vi "TLB Native Dynamic Events ver 0.25.vi"() -> ()   [LabVIEW 2018] (continued)
              tunnel: [w613 State_Type_Definitions."True Stop" ("Enum")] -> w597
              tunnel: [w611 w628] -> w590
              tunnel: w599 -> [w610 _]
              tunnel: w598 -> [w604 _]
              tunnel: [State_Type_Definitions."Idle" ("Enum") State_Type_Definitions."Shutdown" ("Enum")] -> w596
              tunnel: w600 -> [w603 _]
              frame "Start Task 1", Default {
                # ">> WIill proceed to part ii if not manual override >>"
                # ">>If ENABLE or Trigger is set to true>>"
                n263 = Or(x=w603, y=w604) -> (x .or. y?=w605:bool)
                n264 = case shown="True" w603 {
                  tunnel: [w616 w622] -> w611
                  tunnel: w610 -> [w615 w621]
                  frame False {
                    n265 = for {
                      shift-right: [w618] -> w616
                      shift-left: w615 -> [w619]
                      tunnel: string[] ["Z STEPPER CAM HEIGHT", "READ STEPPER VALUES"] ("element") -> [w617] mode=indexing
                      n266 = Enqueue Element(queue=w619, element=w617) -> (queue out=w618:refnum<queue>)  [unwired: 2 in, 2 out]
                    }
                  }
                  frame True {
                    n267 = for {
                      shift-right: [w624] -> w622
                      shift-left: w621 -> [w625]
                      tunnel: string[] ["ARDUINO - ULTRASONIC", "READ ULTRASONIC", "", "", "", ""] -> [w623] mode=indexing
                      n268 = Enqueue Element(queue=w625, element=w623) -> (queue out=w624:refnum<queue>)  [unwired: 2 in, 2 out]
                    }
                  }
                }
                n269 = Select(t=State_Type_Definitions."True Stop" ("Enum"), s=w604, f=State_Type_Definitions."Task 2:Sensor Mode" ("Enum")) -> (s? t:f=w607:T16)
                n270 = Select(t=w607, s=w605, f=State_Type_Definitions."Task 2:Raise Arm" ("Enum")) -> (s? t:f=w613:T16)
              }
              frame "Exit" {
                n271 = for {
                  shift-right: [w631] -> w628
                  shift-left: _ -> [w632]
                  tunnel: string[] ["STOP", "RESET ENCODERS", "RESET YAW", ""] -> [w630] mode=indexing
                  n272 = Enqueue Element(queue=w632, element=w630) -> (queue out=w631:refnum<queue>)  [unwired: 2 in, 2 out]
                }
              }
            }
          }
          frame "Task 2:Sensor Mode" {
            w649 = u8 20 ("y")
            # ">>> yStepper command>>>"
            # ">>Object detected>>"
            n273 = Dequeue Element(queue=w642, timeout in ms (-1)=w641, error in (no error)=w640) -> (element=w650:T8)  [unwired: 3 out]
            n274 = Less?(x=w638, y=w649) -> (x < y?=w648:bool)
            n275 = Less?(x=w637, y=w649) -> (x < y?=w647:bool)
            n276 = Or(x=w648, y=w647) -> (x .or. y?=w633:bool)
            n277 = case shown="\"Start Task 1\", Default" w650 {
              tunnel: w633 -> [w653 _]
              tunnel: [w660 State_Type_Definitions."True Stop" ("Enum")] -> w646
              tunnel: w639 -> [w652 _]
              tunnel: w643 -> [w659 w676]
              tunnel: [w658 w677] -> w645
              tunnel: [State_Type_Definitions."Idle" ("Enum") State_Type_Definitions."Shutdown" ("Enum")] -> w644
              frame "Start Task 1", Default {
                n278 = case shown="False" w653 {
                  tunnel: w659 -> [w663 w670]
                  tunnel: [w664 w669] -> w658
                  frame False {
                    n279 = for {
                      tunnel: string[] ["READ ULTRASONIC", "STOP"] ("element") -> [w665] mode=indexing
                      shift-right: [w667] -> w664
                      shift-left: w663 -> [w666]
                      n280 = Enqueue Element(queue=w666, element=w665) -> (queue out=w667:refnum<queue>)  [unwired: 2 in, 2 out]
                    }
                  }
                  frame True {
                    n281 = for {
                      shift-right: [w672] -> w669
                      shift-left: w670 -> [w673]
                      tunnel: string[] ["RESET ENCODERS", "READ NAVX", "READ ENCODERS"] -> [w671] mode=indexing
                      n282 = Enqueue Element(queue=w673, element=w671) -> (queue out=w672:refnum<queue>)  [unwired: 2 in, 2 out]
                    }
                  }
                }
                n283 = Or(x=w653, y=w652) -> (x .or. y?=w651:bool)
                n284 = Select(t=State_Type_Definitions."True Stop" ("Enum"), s=w652, f=State_Type_Definitions."Task 2:Reverse Mode" ("Enum")) -> (s? t:f=w654:T16)
                n285 = Select(t=w654, s=w651, f=State_Type_Definitions."Task 2:Sensor Mode" ("Enum")) -> (s? t:f=w660:T16)
              }
              frame "Exit" {
                n286 = for {
                  shift-right: [w680] -> w677
                  shift-left: w676 -> [w681]
                  tunnel: string[] ["STOP", "RESET ENCODERS", "RESET YAW", "ARDUINO MODE 0"] -> [w679] mode=indexing
                  n287 = Enqueue Element(queue=w681, element=w679) -> (queue out=w680:refnum<queue>)  [unwired: 2 in, 2 out]
                }
              }
            }
          }
          frame "Task 2:Reverse Mode" {
            # ">>> yStepper command>>>"
            n288 = Dequeue Element(queue=w692, timeout in ms (-1)=w693, error in (no error)=w694) -> (element=w696:T8)  [unwired: 3 out]
            n289 = Less?(x=w686, y=-50.0) -> (x < y?=w684:bool)
            n290 = case shown="\"Start Task 1\", Default" w696 {
              tunnel: [w706 State_Type_Definitions."True Stop" ("Enum")] -> w688
              tunnel: w695 -> [w699 _]
              tunnel: w691 -> [w705 w722]
              tunnel: [w704 w723] -> w687
              tunnel: [State_Type_Definitions."Idle" ("Enum") State_Type_Definitions."Shutdown" ("Enum")] -> w689
              tunnel: w684 -> [w697 _]
              frame "Start Task 1", Default {
                n291 = case shown="True" w697 {
                  tunnel: w705 -> [w709 w716]
                  tunnel: [w710 w715] -> w704
                  frame False {
                    n292 = for {
                      tunnel: string[] ["READ ENCODERS", "REVERSE", "READ NAVX"] ("element") -> [w711] mode=indexing
                      shift-right: [w713] -> w710
                      shift-left: w709 -> [w712]
                      n293 = Enqueue Element(queue=w712, element=w711) -> (queue out=w713:refnum<queue>)  [unwired: 2 in, 2 out]
                    }
                  }
                  frame True {
                    n294 = for {
                      shift-right: [w718] -> w715
                      shift-left: w716 -> [w719]
                      tunnel: string[] ["STOP", "ARDUINO - ULTRASONIC", "READ ULTRASONIC", "RESET ENCODERS"] -> [w717] mode=indexing
                      n295 = Enqueue Element(queue=w719, element=w717) -> (queue out=w718:refnum<queue>)  [unwired: 2 in, 2 out]
                    }
                  }
                }
                n296 = Or(x=w697, y=w699) -> (x .or. y?=w698:bool)
                n297 = Select(t=State_Type_Definitions."True Stop" ("Enum"), s=w699, f=State_Type_Definitions."Task 2:Sensor Mode" ("Enum")) -> (s? t:f=w700:T16)
                n298 = Select(t=w700, s=w698, f=State_Type_Definitions."Task 2:Reverse Mode" ("Enum")) -> (s? t:f=w706:T16)
              }
              frame "Exit" {
                n299 = for {
                  shift-right: [w726] -> w723
                  shift-left: w722 -> [w727]
                  tunnel: string[] ["STOP", "RESET ENCODERS", "RESET YAW", "ARDUINO MODE 0"] -> [w725] mode=indexing
                  n300 = Enqueue Element(queue=w727, element=w725) -> (queue out=w726:refnum<queue>)  [unwired: 2 in, 2 out]
                }
              }
            }
          }
          frame "Task 3" {
            # ">>> Motor control cluster >>>"
            # ">>> yStepper command>>>"
            n301 = Dequeue Element(queue=w743, timeout in ms (-1)=w742, error in (no error)=w741) -> (element=w732:T8)  [unwired: 3 out]
            n302 = Less?(x=w740, y=-160.0) -> (x < y?=w737:bool)
            n303 = Or(x=w737, y=w738) -> (x .or. y?=w733:bool)
            n304 = case shown="\"Start Task 1\", Default" w732 {
              tunnel: w733 -> [w746 _]
              tunnel: [w750 State_Type_Definitions."True Stop" ("Enum")] -> w734
              tunnel: w736 -> [w747 w766]
              tunnel: [w745 w765] -> w735
              tunnel: [State_Type_Definitions."Idle" ("Enum") State_Type_Definitions."Shutdown" ("Enum")] -> w731
              frame "Start Task 1", Default {
                n305 = case shown="False" w746 {
                  tunnel: w747 -> [w753 w759]
                  tunnel: [w752 w757] -> w745
                  frame False {
                    n306 = for {
                      shift-right: [w755] -> w752
                      shift-left: w753 -> [w756]
                      tunnel: string[] ["READ ENCODERS", "R-CW"] ("element") -> [w754] mode=indexing
                      n307 = Enqueue Element(queue=w756, element=w754) -> (queue out=w755:refnum<queue>)  [unwired: 2 in, 2 out]
                    }
                  }
                  frame True {
                    n308 = for {
                      shift-right: [w761] -> w757
                      shift-left: w759 -> [w762]
                      tunnel: string[] ["RESET YAW", "RESET ENCODERS", "STOP", "ARDUINO MODE 0"] -> [w760] mode=indexing
                      n309 = Enqueue Element(queue=w762, element=w760) -> (queue out=w761:refnum<queue>)  [unwired: 2 in, 2 out]
                    }
                  }
                }
                n310 = Select(t=State_Type_Definitions."True Stop" ("Enum"), s=w746, f=State_Type_Definitions."Task 3" ("Enum")) -> (s? t:f=w750:T16)
              }
              frame "Exit" {
                n311 = for {
                  shift-right: [w769] -> w765
                  shift-left: w766 -> [w770]
                  tunnel: string[] ["STOP", "RESET ENCODERS", "RESET YAW", ""] -> [w768] mode=indexing
                  n312 = Enqueue Element(queue=w770, element=w768) -> (queue out=w769:refnum<queue>)  [unwired: 2 in, 2 out]
                }
              }
            }
          }
          frame "Task 4_A" {
            # ">> Stepper height reeached >>"
            # ">>> yStepper command>>>"
            # ">> Manual override >>"
            n313 = Dequeue Element(queue=w784, timeout in ms (-1)=w783, error in (no error)=w782) -> (element=w781:T8)  [unwired: 3 out]
            n314 = Equal?(x=w775, y=u8 60) -> (x = y?=w773:bool)
            n315 = case shown="\"Start Task 1\", Default" w781 {
              tunnel: [w796 State_Type_Definitions."True Stop" ("Enum")] -> w780
              tunnel: [w794 w812] -> w779
              tunnel: w785 -> [w793 w809]
              tunnel: w778 -> [w787 _]
              tunnel: [State_Type_Definitions."Idle" ("Enum") State_Type_Definitions."Shutdown" ("Enum")] -> w777
              tunnel: w773 -> [w786 _]
              frame "Start Task 1", Default {
                # ">> WIill proceed to part ii if not manual override >>"
                # ">>If ENABLE or Trigger is set to true>>"
                n316 = Or(x=w786, y=w787) -> (x .or. y?=w788:bool)
                n317 = case shown="False" w786 {
                  tunnel: [w799 w805] -> w794
                  tunnel: w793 -> [w798 w804]
                  frame False {
                    n318 = for {
                      shift-right: [w801] -> w799
                      shift-left: w798 -> [w802]
                      tunnel: string[] ["Z STEPPER CAM HEIGHT", "READ STEPPER VALUES"] ("element") -> [w800] mode=indexing
                      n319 = Enqueue Element(queue=w802, element=w800) -> (queue out=w801:refnum<queue>)  [unwired: 2 in, 2 out]
                    }
                  }
                  frame True {
                    n320 = for {
                      shift-right: [w807] -> w805
                      shift-left: w804 -> [w808]
                      tunnel: string[] ["ARDUINO - ULTRASONIC", "READ ULTRASONIC", "FORWARD", "", "", ""] -> [w806] mode=indexing
                      n321 = Enqueue Element(queue=w808, element=w806) -> (queue out=w807:refnum<queue>)  [unwired: 2 in, 2 out]
                    }
                  }
                }
                n322 = Select(t=State_Type_Definitions."True Stop" ("Enum"), s=w787, f=State_Type_Definitions."Task 4_B" ("Enum")) -> (s? t:f=w790:T16)
                n323 = Select(t=w790, s=w788, f=State_Type_Definitions."Task 4_A" ("Enum")) -> (s? t:f=w796:T16)
              }
              frame "Exit" {
                n324 = for {
                  shift-right: [w815] -> w812
                  shift-left: w809 -> [w816]
                  tunnel: string[] ["STOP", "RESET ENCODERS", "RESET YAW", ""] -> [w814] mode=indexing
                  n325 = Enqueue Element(queue=w816, element=w814) -> (queue out=w815:refnum<queue>)  [unwired: 2 in, 2 out]
                }
              }
            }
          }
          frame "Task 4_B" {
            w822 = u8 20
            # ">> Path blocked >>"
            # ">>> yStepper command>>>"
            # ">> Manual override >>"
            n326 = Dequeue Element(queue=w831, timeout in ms (-1)=w830, error in (no error)=w829) -> (element=w828:T8)  [unwired: 3 out]
            n327 = Less?(x=w824, y=w822) -> (x < y?=w819:bool)
            n328 = Less?(x=w823, y=w822) -> (x < y?=w820:bool)
            n329 = And(x=w820, y=w819) -> (x .and. y?=w821:bool)
            n330 = case shown="\"Start Task 1\", Default" w828 {
              tunnel: [w845 State_Type_Definitions."True Stop" ("Enum")] -> w833
              tunnel: [w843 w860] -> w834
              tunnel: w827 -> [w842 _]
              tunnel: w832 -> [w836 _]
              tunnel: [State_Type_Definitions."Idle" ("Enum") State_Type_Definitions."Shutdown" ("Enum")] -> w826
              tunnel: w821 -> [w835 _]
              frame "Start Task 1", Default {
                # ">> Manual override forces program to true stop >>"
                # ">>If ENABLE or Trigger is set to true>>"
                n331 = Or(x=w835, y=w836) -> (x .or. y?=w841:bool)
                n332 = case shown="False" w835 {
                  tunnel: [w848 w853] -> w843
                  tunnel: w842 -> [w847 w852]
                  frame False {
                    n333 = for {
                      shift-right: [w850] -> w848
                      shift-left: w847 -> [w851]
                      tunnel: string[] ["FORWARD", "READ ULTRASONIC", "READ NAVX"] ("element") -> [w849] mode=indexing
                      n334 = Enqueue Element(queue=w851, element=w849) -> (queue out=w850:refnum<queue>)  [unwired: 2 in, 2 out]
                    }
                  }
                  frame True {
                    n335 = for {
                      shift-right: [w856] -> w853
                      shift-left: w852 -> [w857]
                      tunnel: string[] ["STOP", "RESET YAW", "RESET ENCODERS", "RESET FLAGS"] -> [w855] mode=indexing
                      n336 = Enqueue Element(queue=w857, element=w855) -> (queue out=w856:refnum<queue>)  [unwired: 2 in, 2 out]
                    }
                  }
                }
                n337 = Select(t=State_Type_Definitions."True Stop" ("Enum"), s=w836, f=State_Type_Definitions."Task 4_C" ("Enum")) -> (s? t:f=w838:T16)
                n338 = Select(t=w838, s=w841, f=State_Type_Definitions."Task 4_B" ("Enum")) -> (s? t:f=w845:T16)
              }
              frame "Exit" {
                n339 = for {
                  shift-right: [w863] -> w860
                  shift-left: _ -> [w864]
                  tunnel: string[] ["STOP", "RESET ENCODERS", "RESET YAW", ""] -> [w862] mode=indexing
                  n340 = Enqueue Element(queue=w864, element=w862) -> (queue out=w863:refnum<queue>)  [unwired: 2 in, 2 out]
                }
              }
            }
          }
          frame "Task 4_C" {
            w876 = u8 20
            # ">> xDistance travelled>>"
            # ">> Path NOT blocked >>"
            # ">>> yStepper command>>>"
            # ">> Manual override >>"
            n341 = Dequeue Element(queue=w886, timeout in ms (-1)=w879, error in (no error)=w878) -> (element=w880:T8)  [unwired: 3 out]
            n342 = Greater?(x=w868, y=w876) -> (0:w874:bool)
            n343 = Greater?(x=w873, y=80.0) -> (0:w871:bool)
            n344 = Greater?(x=w867, y=w876) -> (0:w875:bool)
            n345 = And(x=w875, y=w874) -> (x .and. y?=w870:bool)
            n346 = And(x=w871, y=w870) -> (x .and. y?=w869:bool)
            n347 = case shown="\"Start Task 1\", Default" w880 {
              tunnel: [w897 State_Type_Definitions."True Stop" ("Enum")] -> w883
              tunnel: [w895 w913] -> w882
              tunnel: w885 -> [w894 w910]
              tunnel: w884 -> [w888 _]
              tunnel: [State_Type_Definitions."Idle" ("t") State_Type_Definitions."Shutdown" ("Enum")] -> w881
              tunnel: w869 -> [w887 _]
              frame "Start Task 1", Default {
                # ">> Manual override forces program to true stop >>"
                # ">>If ENABLE or Trigger is set to true>>"
                n348 = Or(x=w887, y=w888) -> (x .or. y?=w893:bool)
                n349 = case shown="False" w887 {
                  tunnel: [w900 w905] -> w895
                  tunnel: w894 -> [w898 w904]
                  frame False {
                    n350 = for {
                      shift-right: [w902] -> w900
                      shift-left: w898 -> [w903]
                      tunnel: string[] ["RIGHT", "READ NAVX", "READ ENCODERS", "READ ULTRASONIC"] ("element") -> [w901] mode=indexing
                      n351 = Enqueue Element(queue=w903, element=w901) -> (queue out=w902:refnum<queue>)  [unwired: 2 in, 2 out]
                    }
                  }
                  frame True {
                    n352 = for {
                      shift-right: [w908] -> w905
                      shift-left: w904 -> [w909]
                      tunnel: string[] ["STOP", "RESET YAW", "RESET ENCODERS", "ARDUINO - ULTRASONIC"] -> [w907] mode=indexing
                      n353 = Enqueue Element(queue=w909, element=w907) -> (queue out=w908:refnum<queue>)  [unwired: 2 in, 2 out]
                    }
                  }
                }
                n354 = Select(t=State_Type_Definitions."True Stop" ("Enum"), s=w888, f=State_Type_Definitions."Task 4_D" ("Enum")) -> (s? t:f=w889:T16)
                n355 = Select(t=w889, s=w893, f=State_Type_Definitions."Task 4_C" ("Enum")) -> (s? t:f=w897:T16)
              }
              frame "Exit" {
                n356 = for {
                  shift-right: [w916] -> w913
                  shift-left: w910 -> [w917]
                  tunnel: string[] ["STOP", "RESET ENCODERS", "RESET YAW", ""] -> [w915] mode=indexing
                  n357 = Enqueue Element(queue=w917, element=w915) -> (queue out=w916:refnum<queue>)  [unwired: 2 in, 2 out]
                }
              }
            }
          }
          frame "Task 4_D" {
            w940 = u8 20
            # ">>> Motor control cluster >>>"
            # ">> Line detected >>"
            # ">> yDistance travelled>>"
            # ">> Path blocked >>"
            # ">>> yStepper command>>>"
            # ">> Manual override >>"
            n358 = Less?(x=w925, y=w940) -> (x < y?=w938:bool)
            n359 = Greater?(x=w929, y=200.0) -> (0:w936:bool)
            n360 = Less?(x=w924, y=w940) -> (x < y?=w939:bool)
            n361 = And(x=w939, y=w938) -> (x .and. y?=w935:bool)
            n362 = Dequeue Element(queue=w932, timeout in ms (-1)=w931, error in (no error)=w930) -> (element=w941:T8)  [unwired: 3 out]
            n363 = Or(x=w936, y=w935) -> (x .or. y?=w919:bool)
            n364 = And(x=w920, y=w919) -> (x .and. y?=w918:bool)
            n365 = case shown="\"Start Task 1\", Default" w941 {
              tunnel: [w952 State_Type_Definitions."True Stop" ("Enum")] -> w928
              tunnel: [w950 w968] -> w926
              tunnel: w933 -> [w949 w965]
              tunnel: w934 -> [w943 _]
              tunnel: [State_Type_Definitions."Idle" ("t") State_Type_Definitions."Shutdown" ("Enum")] -> w927
              tunnel: w918 -> [w942 _]
              frame "Start Task 1", Default {
                # ">> Manual override forces program to true stop >>"
                # ">>If ENABLE or Trigger is set to true>>"
                n366 = Or(x=w942, y=w943) -> (x .or. y?=w948:bool)
                n367 = case shown="False" w942 {
                  tunnel: [w955 w960] -> w950
                  tunnel: w949 -> [w953 w959]
                  frame False {
                    n368 = for {
                      shift-right: [w957] -> w955
                      shift-left: w953 -> [w958]
                      tunnel: string[] ["FORWARD", "READ NAVX", "READ ENCODERS", "READ ULTRASONIC", "READ LINE SENSOR"] ("element") -> [w956] mode=indexing
                      n369 = Enqueue Element(queue=w958, element=w956) -> (queue out=w957:refnum<queue>)  [unwired: 2 in, 2 out]
                    }
                  }
                  frame True {
                    n370 = for {
                      shift-right: [w963] -> w960
                      shift-left: w959 -> [w964]
                      tunnel: string[] ["STOP", "RESET YAW", "RESET ENCODERS", "RESET FLAGS"] -> [w962] mode=indexing
                      n371 = Enqueue Element(queue=w964, element=w962) -> (queue out=w963:refnum<queue>)  [unwired: 2 in, 2 out]
                    }
                  }
                }
                n372 = Select(t=State_Type_Definitions."True Stop" ("Enum"), s=w943, f=State_Type_Definitions."True Stop" ("Enum")) -> (s? t:f=w944:T16)
                n373 = Select(t=w944, s=w948, f=State_Type_Definitions."Task 4_D" ("Enum")) -> (s? t:f=w952:T16)
              }
              frame "Exit" {
                n374 = for {
                  shift-right: [w971] -> w968
                  shift-left: w965 -> [w972]
                  tunnel: string[] ["STOP", "RESET ENCODERS", "RESET YAW", ""] -> [w970] mode=indexing
                  n375 = Enqueue Element(queue=w972, element=w970) -> (queue out=w971:refnum<queue>)  [unwired: 2 in, 2 out]
                }
              }
            }
          }
          frame "Task 5A" {
            # "Stays in Task 5_A until stepper reaches desired \nheight"
            # ">>> Motor control cluster >>>"
            # ">>> yStepper command>>>"
            # ">> Manual override >>"
            n376 = Dequeue Element(queue=w983, timeout in ms (-1)=w982, error in (no error)=w984) -> (element=w981:T8)  [unwired: 3 out]
            n377 = Equal?(x=w980, y=u8 1) -> (x = y?=w978:bool)
            n378 = case shown="\"Start Task 1\", Default" w981 {
              tunnel: [w994 State_Type_Definitions."True Stop" ("Enum")] -> w985
              tunnel: [w997 w1014] -> w986
              tunnel: [State_Type_Definitions."Idle" ("Enum") State_Type_Definitions."Shutdown" ("Enum")] -> w987
              tunnel: w978 -> [w993 _]
              tunnel: w977 -> [w992 _]
              tunnel: w976 -> [w988 w1011]
              frame "Start Task 1", Default {
                # "T: Go back to idle, F: Continue with task\""
                # ">> Manual override >>"
                n379 = case shown="True" w993 {
                  tunnel: [w1001 w1007] -> w997
                  tunnel: w988 -> [w999 w1005]
                  frame False {
                    n380 = for {
                      tunnel: string[] ["Z STEPPER GRAB HEIGHT", "READ STEPPER VALUES"] ("element") -> [w1002] mode=indexing
                      shift-right: [w1004] -> w1001
                      shift-left: w999 -> [w1003]
                      n381 = Enqueue Element(queue=w1003, element=w1002) -> (queue out=w1004:refnum<queue>)  [unwired: 2 in, 2 out]
                    }
                  }
                  frame True {
                    n382 = for {
                      shift-right: [w1009] -> w1007
                      shift-left: w1005 -> [w1010]
                      tunnel: string[] ["SET TIMER 2", "", ""] -> [w1008] mode=indexing
                      n383 = Enqueue Element(queue=w1010, element=w1008) -> (queue out=w1009:refnum<queue>)  [unwired: 2 in, 2 out]
                    }
                  }
                }
                n384 = Or(x=w993, y=w992) -> (x .or. y?=w995:bool)
                n385 = Select(t=State_Type_Definitions."True Stop" ("Enum"), s=w992, f=State_Type_Definitions."Task 5B" ("Enum")) -> (s? t:f=w989:T16)
                n386 = Select(t=w989, s=w995, f=State_Type_Definitions."Task 5A" ("Enum")) -> (s? t:f=w994:T16)
              }
              frame "Exit" {
                n387 = for {
                  shift-right: [w1017] -> w1014
                  shift-left: w1011 -> [w1018]
                  tunnel: string[] ["STOP", "RESET ENCODERS", "RESET YAW", "ARDUINO MODE 0"] -> [w1016] mode=indexing
                  n388 = Enqueue Element(queue=w1018, element=w1016) -> (queue out=w1017:refnum<queue>)  [unwired: 2 in, 2 out]
                }
              }
            }
          }
          frame "Task 5B" {
            # ">>> yStepper command>>>"
            n389 = Dequeue Element(queue=w1025, timeout in ms (-1)=w1024, error in (no error)=w1026) -> (element=w1023:T8)  [unwired: 3 out]
            n390 = case shown="\"Start Task 1\", Default" w1023 {
              tunnel: [w1038 State_Type_Definitions."True Stop" ("Enum")] -> w1028
              tunnel: [w1041 w1058] -> w1027
              tunnel: [State_Type_Definitions."Idle" ("Enum") State_Type_Definitions."Shutdown" ("Enum")] -> w1029
              tunnel: w1031 -> [w1037 _]
              tunnel: w1030 -> [w1033 w1055]
              tunnel: w1019 -> [w1032 _]
              frame "Start Task 1", Default {
                # "T: Go back to idle, F: Continue with task\""
                # ">> Manual override >>"
                n391 = case shown="True" w1032 {
                  tunnel: [w1045 w1051] -> w1041
                  tunnel: w1033 -> [w1043 w1049]
                  frame False {
                    n392 = for {
                      tunnel: string[] ["CLOSE CLAW", "START TIMER", ""] ("element") -> [w1046] mode=indexing
                      shift-right: [w1048] -> w1045
                      shift-left: w1043 -> [w1047]
                      n393 = Enqueue Element(queue=w1047, element=w1046) -> (queue out=w1048:refnum<queue>)  [unwired: 2 in, 2 out]
                    }
                  }
                  frame True {
                    n394 = for {
                      shift-right: [w1053] -> w1051
                      shift-left: w1049 -> [w1054]
                      tunnel: string[] ["STOP", "", "", ""] -> [w1052] mode=indexing
                      n395 = Enqueue Element(queue=w1054, element=w1052) -> (queue out=w1053:refnum<queue>)  [unwired: 2 in, 2 out]
                    }
                  }
                }
                n396 = Or(x=w1032, y=w1037) -> (x .or. y?=w1039:bool)
                n397 = Select(t=State_Type_Definitions."True Stop" ("Enum"), s=w1037, f=State_Type_Definitions."Task 5C" ("Enum")) -> (s? t:f=w1034:T16)
                n398 = Select(t=w1034, s=w1039, f=State_Type_Definitions."Task 5B" ("Enum")) -> (s? t:f=w1038:T16)
              }
              frame "Exit" {
                n399 = for {
                  shift-right: [w1061] -> w1058
                  shift-left: w1055 -> [w1062]
                  tunnel: string[] ["STOP", "RESET ENCODERS", "RESET YAW", "ARDUINO MODE 0"] -> [w1060] mode=indexing
                  n400 = Enqueue Element(queue=w1062, element=w1060) -> (queue out=w1061:refnum<queue>)  [unwired: 2 in, 2 out]
                }
              }
            }
          }
          frame "Task 5C" {
            # ">>> Motor control cluster >>>"
            # ">>> yStepper command>>>"
            # ">> Manual override >>"
            n401 = Equal?(x=w1065, y=u8 60) -> (x = y?=w1063:bool)
            n402 = Dequeue Element(queue=w1075, timeout in ms (-1)=w1074, error in (no error)=w1073) -> (element=w1072:T8)  [unwired: 3 out]
            n403 = case shown="\"Start Task 1\", Default" w1072 {
              tunnel: [w1084 State_Type_Definitions."True Stop" ("Enum")] -> w1077
              tunnel: [w1087 w1104] -> w1070
              tunnel: [State_Type_Definitions."Idle" ("Enum") State_Type_Definitions."Shutdown" ("Enum")] -> w1069
              tunnel: w1071 -> [w1078 _]
              tunnel: w1076 -> [w1083 w1101]
              tunnel: w1063 -> [w1082 _]
              frame "Start Task 1", Default {
                # ">> Is time up? >>"
                # "Determines if object is in range to pick up"
                # ">> Manual override >>"
                n404 = case shown="True" w1082 {
                  tunnel: [w1091 w1097] -> w1087
                  tunnel: w1083 -> [w1089 w1095]
                  frame False {
                    n405 = for {
                      tunnel: string[] ["Z STEPPER CAM HEIGHT", "READ STEPPER VALUES"] ("element") -> [w1092] mode=indexing
                      shift-right: [w1094] -> w1091
                      shift-left: w1089 -> [w1093]
                      n406 = Enqueue Element(queue=w1093, element=w1092) -> (queue out=w1094:refnum<queue>)  [unwired: 2 in, 2 out]
                    }
                  }
                  frame True {
                    n407 = for {
                      shift-right: [w1099] -> w1097
                      shift-left: w1095 -> [w1100]
                      tunnel: string[] ["SET TIMER 5", "", ""] -> [w1098] mode=indexing
                      n408 = Enqueue Element(queue=w1100, element=w1098) -> (queue out=w1099:refnum<queue>)  [unwired: 2 in, 2 out]
                    }
                  }
                }
                n409 = Or(x=w1082, y=w1078) -> (x .or. y?=w1085:bool)
                n410 = Select(t=State_Type_Definitions."True Stop" ("Enum"), s=w1078, f=State_Type_Definitions."Task 5D" ("Enum")) -> (s? t:f=w1080:T16)
                n411 = Select(t=w1080, s=w1085, f=State_Type_Definitions."Task 5C" ("Enum")) -> (s? t:f=w1084:T16)
              }
              frame "Exit" {
                n412 = for {
                  shift-right: [w1107] -> w1104
                  shift-left: w1101 -> [w1108]
                  tunnel: string[] ["STOP", "RESET ENCODERS", "RESET YAW", "ARDUINO MODE 0"] -> [w1106] mode=indexing
                  n413 = Enqueue Element(queue=w1108, element=w1106) -> (queue out=w1107:refnum<queue>)  [unwired: 2 in, 2 out]
                }
              }
            }
          }
          frame "Task 5D" {
            # ">>> yStepper command>>>"
            n414 = Dequeue Element(queue=w1116, timeout in ms (-1)=w1115, error in (no error)=w1114) -> (element=w1113:T8)  [unwired: 3 out]
            n415 = case shown="\"Start Task 1\", Default" w1113 {
              tunnel: [w1128 State_Type_Definitions."True Stop" ("Enum")] -> w1120
              tunnel: [w1131 w1148] -> w1119
              tunnel: [State_Type_Definitions."Idle" ("Enum") State_Type_Definitions."Shutdown" ("Enum")] -> w1121
              tunnel: w1117 -> [w1127 _]
              tunnel: w1118 -> [w1123 w1145]
              tunnel: w1111 -> [w1122 _]
              frame "Start Task 1", Default {
                # ">> T: Breaks out of state loop; F: Stays in loop>>"
                # ">> Manual override >>"
                # ">> Checks if time is up>>"
                # "Stays in Task 5D until the object is detected"
                # "T: Go back to idle, F: Continue with task\""
                # ">> Manual override >>"
                n416 = case shown="False" w1122 {
                  tunnel: [w1135 w1141] -> w1131
                  tunnel: w1123 -> [w1133 w1139]
                  frame False {
                    n417 = for {
                      tunnel: string[] ["START TIMER", "OPEN CLAW", ""] ("element") -> [w1136] mode=indexing
                      shift-right: [w1138] -> w1135
                      shift-left: w1133 -> [w1137]
                      n418 = Enqueue Element(queue=w1137, element=w1136) -> (queue out=w1138:refnum<queue>)  [unwired: 2 in, 2 out]
                    }
                  }
                  frame True {
                    n419 = for {
                      shift-right: [w1143] -> w1141
                      shift-left: w1139 -> [w1144]
                      tunnel: string[] ["CAM CLOSE", "", ""] -> [w1142] mode=indexing
                      n420 = Enqueue Element(queue=w1144, element=w1142) -> (queue out=w1143:refnum<queue>)  [unwired: 2 in, 2 out]
                    }
                  }
                }
                n421 = Or(x=w1122, y=w1127) -> (x .or. y?=w1129:bool)
                n422 = Select(t=State_Type_Definitions."True Stop" ("Enum"), s=w1127, f=State_Type_Definitions."True Stop" ("Enum")) -> (s? t:f=w1124:T16)
                n423 = Select(t=w1124, s=w1129, f=State_Type_Definitions."Task 5D" ("Enum")) -> (s? t:f=w1128:T16)
              }
              frame "Exit" {
                n424 = for {
                  shift-right: [w1151] -> w1148
                  shift-left: w1145 -> [w1152]
                  tunnel: string[] ["STOP", "RESET ENCODERS", "RESET YAW", "ARDUINO MODE 0"] -> [w1150] mode=indexing
                  n425 = Enqueue Element(queue=w1152, element=w1150) -> (queue out=w1151:refnum<queue>)  [unwired: 2 in, 2 out]
                }
              }
            }
          }
          frame "Task 5E: POSITION ARM" {
            # ">>> yStepper command>>>"
            n426 = Dequeue Element(queue=w1166, timeout in ms (-1)=w1167, error in (no error)=w1168) -> (element=w1170:T8)  [unwired: 3 out]
            n427 = formula code="if (pos < 100)\ny = 41;\n\nelse if (pos >= 100 && pos <= 140)\ny = 30;\n\nelse if (pos >= 141 && pos <= 170)\ny = 25;\n\nelse if (pos >= 171 &&pos <= 180) \ny = 20;\n\nelse if (pos >= 181&& pos <= 200)\ny = 15;\n\nelse if (pos >= 201 && pos <= 230)\ny = 10;\n\nelse if (pos >= 231 && pos <= 320)\ny = 8;\n\nelse if (pos > 320)\ny = 0;"("pos"=w1158) -> ("y"=w1161:dbl)
            n428 = To Unsigned Byte Integer(number=w1161) -> (unsigned 8bit integer=w1156:u8)
            n429 = Equal?(x=w1157, y=w1156) -> (x = y?=w1155:bool)
            n430 = case shown="\"Start Task 1\", Default" w1170 {
              tunnel: [w1177 State_Type_Definitions."True Stop" ("Enum")] -> w1164
              tunnel: [w1180 w1197] -> w1162
              tunnel: [State_Type_Definitions."Idle" ("Enum") State_Type_Definitions."Shutdown" ("Enum")] -> w1163
              tunnel: w1169 -> [w1176 _]
              tunnel: w1165 -> [w1172 w1194]
              tunnel: w1155 -> [w1171 _]
              frame "Start Task 1", Default {
                # ">> T: Breaks out of state loop; F: Stays in loop>>"
                # ">> Manual override >>"
                # ">> Checks if time is up>>"
                # "Stays in Task 5D until the object is detected"
                # "T: Go back to idle, F: Continue with task\""
                # ">> Manual override >>"
                n431 = case shown="False" w1171 {
                  tunnel: [w1184 w1190] -> w1180
                  tunnel: w1172 -> [w1182 w1188]
                  frame False {
                    n432 = for {
                      tunnel: string[] ["READ STEPPER VALUES", "Y STEPPER CONTROL", ""] ("element") -> [w1185] mode=indexing
                      shift-right: [w1187] -> w1184
                      shift-left: w1182 -> [w1186]
                      n433 = Enqueue Element(queue=w1186, element=w1185) -> (queue out=w1187:refnum<queue>)  [unwired: 2 in, 2 out]
                    }
                  }
                  frame True {
                    n434 = for {
                      shift-right: [w1192] -> w1190
                      shift-left: w1188 -> [w1193]
                      tunnel: string[] ["CAM CLOSE", "DISPOSE BUFFERS", ""] -> [w1191] mode=indexing
                      n435 = Enqueue Element(queue=w1193, element=w1191) -> (queue out=w1192:refnum<queue>)  [unwired: 2 in, 2 out]
                    }
                  }
                }
                n436 = Or(x=w1171, y=w1176) -> (x .or. y?=w1178:bool)
                n437 = Select(t=State_Type_Definitions."True Stop" ("Enum"), s=w1176, f=State_Type_Definitions."Task 5F: ARM GRAB HEIGHT" ("Enum")) -> (s? t:f=w1173:T16)
                n438 = Select(t=w1173, s=w1178, f=State_Type_Definitions."Task 5E: POSITION ARM" ("Enum")) -> (s? t:f=w1177:T16)
              }
              frame "Exit" {
                n439 = for {
                  shift-right: [w1200] -> w1197
                  shift-left: w1194 -> [w1201]
                  tunnel: string[] ["STOP", "RESET ENCODERS", "RESET YAW", "ARDUINO MODE 0"] -> [w1199] mode=indexing
                  n440 = Enqueue Element(queue=w1201, element=w1199) -> (queue out=w1200:refnum<queue>)  [unwired: 2 in, 2 out]
                }
              }
            }
            n441 = Bundle By Name(cluster=w1160, "yStepper desired"=w1156) -> (w1159:T18)
          }
          frame "Task 5F: ARM GRAB HEIGHT" {
            # ">>> Motor control cluster >>>"
            # ">>> yStepper command>>>"
            # ">> Manual override >>"
            n442 = Dequeue Element(queue=w1212, timeout in ms (-1)=w1211, error in (no error)=w1213) -> (element=w1210:T8)  [unwired: 3 out]
            n443 = Equal?(x=w1209, y=u8 1) -> (x = y?=w1207:bool)
            n444 = case shown="\"Start Task 1\", Default" w1210 {
              tunnel: [w1223 State_Type_Definitions."True Stop" ("Enum")] -> w1214
              tunnel: [w1226 w1243] -> w1215
              tunnel: [State_Type_Definitions."Idle" ("Enum") State_Type_Definitions."Shutdown" ("Enum")] -> w1216
              tunnel: w1207 -> [w1222 _]
              tunnel: w1206 -> [w1221 _]
              tunnel: w1205 -> [w1217 w1240]
              frame "Start Task 1", Default {
                # "Stays in Task 5F until stepper reaches desired \nheight"
                # "T: Go back to idle, F: Continue with task\""
                # ">> Manual override >>"
                n445 = case shown="True" w1222 {
                  tunnel: [w1230 w1236] -> w1226
                  tunnel: w1217 -> [w1228 w1234]
                  frame False {
                    n446 = for {
                      tunnel: string[] ["Z STEPPER GRAB HEIGHT", "READ STEPPER VALUES"] ("element") -> [w1231] mode=indexing
                      shift-right: [w1233] -> w1230
                      shift-left: w1228 -> [w1232]
                      n447 = Enqueue Element(queue=w1232, element=w1231) -> (queue out=w1233:refnum<queue>)  [unwired: 2 in, 2 out]
                    }
                  }
                  frame True {
                    n448 = for {
                      shift-right: [w1238] -> w1236
                      shift-left: w1234 -> [w1239]
                      tunnel: string[] ["SET TIMER 5", "CLOSE CLAW", ""] -> [w1237] mode=indexing
                      n449 = Enqueue Element(queue=w1239, element=w1237) -> (queue out=w1238:refnum<queue>)  [unwired: 2 in, 2 out]
                    }
                  }
                }
                n450 = Or(x=w1222, y=w1221) -> (x .or. y?=w1224:bool)
                n451 = Select(t=State_Type_Definitions."True Stop" ("Enum"), s=w1221, f=State_Type_Definitions."Task 5G: CLOSE CLAW" ("Enum")) -> (s? t:f=w1218:T16)
                n452 = Select(t=w1218, s=w1224, f=State_Type_Definitions."Task 5F: ARM GRAB HEIGHT" ("Enum")) -> (s? t:f=w1223:T16)
              }
              frame "Exit" {
                n453 = for {
                  shift-right: [w1246] -> w1243
                  shift-left: w1240 -> [w1247]
                  tunnel: string[] ["STOP", "RESET ENCODERS", "RESET YAW", "ARDUINO MODE 0"] -> [w1245] mode=indexing
                  n454 = Enqueue Element(queue=w1247, element=w1245) -> (queue out=w1246:refnum<queue>)  [unwired: 2 in, 2 out]
                }
              }
            }
          }
          frame "Task 5G: CLOSE CLAW" {
            # ">>> yStepper command>>>"
            # ">> Manual override >>"
            n455 = Dequeue Element(queue=w1258, timeout in ms (-1)=w1257, error in (no error)=w1256) -> (element=w1255:T8)  [unwired: 3 out]
            n456 = case shown="\"Start Task 1\", Default" w1255 {
              tunnel: [w1267 State_Type_Definitions."True Stop" ("Enum")] -> w1260
              tunnel: [w1270 w1287] -> w1253
              tunnel: [State_Type_Definitions."Idle" ("Enum") State_Type_Definitions."Shutdown" ("Enum")] -> w1252
              tunnel: w1254 -> [w1261 _]
              tunnel: w1259 -> [w1266 w1284]
              tunnel: w1250 -> [w1265 _]
              frame "Start Task 1", Default {
                # ">> Is time up? >>"
                # "Determines if object is in range to pick up"
                # ">> Manual override >>"
                n457 = case shown="True" w1265 {
                  tunnel: [w1274 w1280] -> w1270
                  tunnel: w1266 -> [w1272 w1278]
                  frame False {
                    n458 = for {
                      tunnel: string[] ["CLOSE CLAW", "START TIMER"] ("element") -> [w1275] mode=indexing
                      shift-right: [w1277] -> w1274
                      shift-left: w1272 -> [w1276]
                      n459 = Enqueue Element(queue=w1276, element=w1275) -> (queue out=w1277:refnum<queue>)  [unwired: 2 in, 2 out]
                    }
                  }
                  frame True {
                    n460 = for {
                      shift-right: [w1282] -> w1280
                      shift-left: w1278 -> [w1283]
                      tunnel: string[] ["READ STEPPER VALUES", "", ""] -> [w1281] mode=indexing
                      n461 = Enqueue Element(queue=w1283, element=w1281) -> (queue out=w1282:refnum<queue>)  [unwired: 2 in, 2 out]
                    }
                  }
                }
                n462 = Or(x=w1265, y=w1261) -> (x .or. y?=w1268:bool)
                n463 = Select(t=State_Type_Definitions."True Stop" ("Enum"), s=w1261, f=State_Type_Definitions."Task 5H: RAISE ARM" ("Enum")) -> (s? t:f=w1263:T16)
                n464 = Select(t=w1263, s=w1268, f=State_Type_Definitions."Task 5G: CLOSE CLAW" ("Enum")) -> (s? t:f=w1267:T16)
              }
              frame "Exit" {
                n465 = for {
                  shift-right: [w1290] -> w1287
                  shift-left: w1284 -> [w1291]
                  tunnel: string[] ["STOP", "RESET ENCODERS", "RESET YAW", "ARDUINO MODE 0"] -> [w1289] mode=indexing
                  n466 = Enqueue Element(queue=w1291, element=w1289) -> (queue out=w1290:refnum<queue>)  [unwired: 2 in, 2 out]
                }
              }
            }
          }
          frame "Task 5H: RAISE ARM" {
            # ">>> yStepper command>>>"
            # ">> Manual override >>"
            n467 = Dequeue Element(queue=w1302, timeout in ms (-1)=w1301, error in (no error)=w1303) -> (element=w1300:T8)  [unwired: 3 out]
            n468 = Equal?(x=w1299, y=u8 60) -> (x = y?=w1297:bool)
            n469 = case shown="\"Start Task 1\", Default" w1300 {
              tunnel: [w1313 State_Type_Definitions."True Stop" ("Enum")] -> w1304
              tunnel: [w1316 w1333] -> w1305
              tunnel: [State_Type_Definitions."Idle" ("Enum") State_Type_Definitions."Shutdown" ("Enum")] -> w1306
              tunnel: w1297 -> [w1312 _]
              tunnel: w1296 -> [w1311 _]
              tunnel: w1295 -> [w1307 w1330]
              frame "Start Task 1", Default {
                # "Stays in Task 5_A until stepper reaches desired \nheight"
                # "T: Go back to idle, F: Continue with task\""
                # ">> Manual override >>"
                n470 = case shown="False" w1312 {
                  tunnel: [w1320 w1326] -> w1316
                  tunnel: w1307 -> [w1318 w1324]
                  frame False {
                    n471 = for {
                      tunnel: string[] ["Z STEPPER CAM HEIGHT", "READ STEPPER VALUES"] ("element") -> [w1321] mode=indexing
                      shift-right: [w1323] -> w1320
                      shift-left: w1318 -> [w1322]
                      n472 = Enqueue Element(queue=w1322, element=w1321) -> (queue out=w1323:refnum<queue>)  [unwired: 2 in, 2 out]
                    }
                  }
                  frame True {
                    n473 = for {
                      shift-right: [w1328] -> w1326
                      shift-left: w1324 -> [w1329]
                      tunnel: string[] ["ARDUINO - ULTRASONIC", "READ ULTRASONIC", ""] -> [w1327] mode=indexing
                      n474 = Enqueue Element(queue=w1329, element=w1327) -> (queue out=w1328:refnum<queue>)  [unwired: 2 in, 2 out]
                    }
                  }
                }
                n475 = Or(x=w1312, y=w1311) -> (x .or. y?=w1314:bool)
                n476 = Select(t=State_Type_Definitions."True Stop" ("Enum"), s=w1311, f=State_Type_Definitions."True Stop" ("Enum")) -> (s? t:f=w1308:T16)
                n477 = Select(t=w1308, s=w1314, f=State_Type_Definitions."Task 5H: RAISE ARM" ("Enum")) -> (s? t:f=w1313:T16)
              }
              frame "Exit" {
                n478 = for {
                  shift-right: [w1336] -> w1333
                  shift-left: w1330 -> [w1337]
                  tunnel: string[] ["STOP", "RESET ENCODERS", "RESET YAW", "ARDUINO MODE 0"] -> [w1335] mode=indexing
                  n479 = Enqueue Element(queue=w1337, element=w1335) -> (queue out=w1336:refnum<queue>)  [unwired: 2 in, 2 out]
                }
              }
            }
          }
          frame "Task 6_A" {
            # ">>> yStepper command>>>"
            n480 = Dequeue Element(queue=w1347, timeout in ms (-1)=w1346, error in (no error)=w1345) -> (element=w1352:T8)  [unwired: 3 out]
            n481 = Equal?(x=w1343, y=u8 60) -> (x = y?=w1342:bool)
            n482 = case shown="\"Start Task 1\", Default" w1352 {
              tunnel: [w1359 State_Type_Definitions."True Stop" ("Enum")] -> w1350
              tunnel: [w1358 w1376] -> w1349
              tunnel: [State_Type_Definitions."Idle" ("Enum") State_Type_Definitions."Shutdown" ("Enum")] -> w1351
              tunnel: w1348 -> [w1354 _]
              tunnel: w1344 -> [w1356 _]
              tunnel: w1342 -> [w1353 _]
              frame "Start Task 1", Default {
                n483 = case shown="False" w1353 {
                  tunnel: [w1364 w1370] -> w1358
                  tunnel: w1356 -> [w1362 w1368]
                  frame False {
                    n484 = for {
                      tunnel: string[] ["Z STEPPER CAM HEIGHT", "READ STEPPER VALUES"] ("element") -> [w1365] mode=indexing
                      shift-right: [w1367] -> w1364
                      shift-left: w1362 -> [w1366]
                      n485 = Enqueue Element(queue=w1366, element=w1365) -> (queue out=w1367:refnum<queue>)  [unwired: 2 in, 2 out]
                    }
                  }
                  frame True {
                    n486 = for {
                      shift-right: [w1372] -> w1370
                      shift-left: w1368 -> [w1373]
                      tunnel: string[] ["CAM ACQ", "OPEN LOG CAM"] -> [w1371] mode=indexing
                      n487 = Enqueue Element(queue=w1373, element=w1371) -> (queue out=w1372:refnum<queue>)  [unwired: 2 in, 2 out]
                    }
                  }
                }
                n488 = Or(x=w1353, y=w1354) -> (x .or. y?=w1355:bool)
                n489 = Select(t=State_Type_Definitions."Task 6_B" ("Enum"), s=w1355, f=State_Type_Definitions."Task 6_A" ("Enum")) -> (s? t:f=w1359:T16)
              }
              frame "Exit" {
                n490 = for {
                  shift-right: [w1379] -> w1376
                  shift-left: _ -> [w1380]
                  tunnel: string[] ["STOP", "RESET ENCODERS", "RESET YAW", "ARDUINO MODE 0"] -> [w1378] mode=indexing
                  n491 = Enqueue Element(queue=w1380, element=w1378) -> (queue out=w1379:refnum<queue>)  [unwired: 2 in, 2 out]
                }
              }
            }
          }
          frame "Task 6_B" {
            # ">>> yStepper command>>>"
            n492 = Dequeue Element(queue=w1392, timeout in ms (-1)=w1390, error in (no error)=w1391) -> (element=w1389:T8)  [unwired: 3 out]
            n493 = case shown="\"Start Task 1\", Default" w1389 {
              tunnel: [w1399 State_Type_Definitions."True Stop" ("Enum")] -> w1385
              tunnel: [w1398 w1417] -> w1393
              tunnel: [State_Type_Definitions."Idle" ("Enum") State_Type_Definitions."Shutdown" ("Enum")] -> w1386
              tunnel: w1388 -> [w1394 _]
              tunnel: w1387 -> [w1396 _]
              tunnel: w1384 -> [w1395 w1414]
              frame "Start Task 1", Default {
                # ">> Manual override >>"
                n494 = case shown="False" w1396 {
                  tunnel: [w1404 w1410] -> w1398
                  tunnel: w1395 -> [w1403 w1408]
                  frame False {
                    n495 = for {
                      shift-right: [w1407] -> w1404
                      shift-left: w1403 -> [w1406]
                      tunnel: string[] ["CAM ACQ", "PROCESS IMAGE", "OPEN CLAW"] -> [w1405] mode=indexing
                      n496 = Enqueue Element(queue=w1406, element=w1405) -> (queue out=w1407:refnum<queue>)  [unwired: 2 in, 2 out]
                    }
                  }
                  frame True {
                    n497 = for {
                      shift-right: [w1412] -> w1410
                      shift-left: w1408 -> [w1413]
                      tunnel: string[] ["CAM ACQ", "PROCESS IMAGE", "CLOSE CLAW"] -> [w1411] mode=indexing
                      n498 = Enqueue Element(queue=w1413, element=w1411) -> (queue out=w1412:refnum<queue>)  [unwired: 2 in, 2 out]
                    }
                  }
                }
                n499 = Select(t=State_Type_Definitions."True Stop" ("Enum"), s=w1394, f=State_Type_Definitions."Task 6_B" ("Enum")) -> (s? t:f=w1399:T16)
              }
              frame "Exit" {
                # ">> State after true stop >>"
                # ">> Goes to true stop >>"
                n500 = for {
                  shift-right: [w1420] -> w1417
                  shift-left: w1414 -> [w1421]
                  tunnel: string[] ["STOP", "RESET ENCODERS", "RESET YAW", ""] -> [w1419] mode=indexing
                  n501 = Enqueue Element(queue=w1421, element=w1419) -> (queue out=w1420:refnum<queue>)  [unwired: 2 in, 2 out]
                }
              }
            }
          }
          frame "Task 7" {
          }
          frame "Task 8A: RAISE ARM" {
            # ">>> Motor control cluster >>>"
            # ">>> yStepper command>>>"
            # ">> Manual override >>"
            n502 = Dequeue Element(queue=w1438, timeout in ms (-1)=w1437, error in (no error)=w1439) -> (element=w1436:T8)  [unwired: 3 out]
            n503 = Equal?(x=w1435, y=u8 60) -> (x = y?=w1433:bool)
            n504 = case shown="\"Start Task 1\", Default" w1436 {
              tunnel: [w1449 State_Type_Definitions."True Stop" ("Enum")] -> w1440
              tunnel: [w1452 w1469] -> w1441
              tunnel: [State_Type_Definitions."Idle" ("Enum") State_Type_Definitions."Shutdown" ("Enum")] -> w1442
              tunnel: w1433 -> [w1448 _]
              tunnel: w1432 -> [w1447 _]
              tunnel: w1431 -> [w1443 w1466]
              frame "Start Task 1", Default {
                # "Stays in Task 5_A until stepper reaches desired \nheight"
                # "T: Go back to idle, F: Continue with task\""
                # ">> Manual override >>"
                n505 = case shown="False" w1448 {
                  tunnel: [w1456 w1462] -> w1452
                  tunnel: w1443 -> [w1454 w1460]
                  frame False {
                    n506 = for {
                      tunnel: string[] ["Z STEPPER CAM HEIGHT", "READ STEPPER VALUES"] ("element") -> [w1457] mode=indexing
                      shift-right: [w1459] -> w1456
                      shift-left: w1454 -> [w1458]
                      n507 = Enqueue Element(queue=w1458, element=w1457) -> (queue out=w1459:refnum<queue>)  [unwired: 2 in, 2 out]
                    }
                  }
                  frame True {
                    n508 = for {
                      shift-right: [w1464] -> w1462
                      shift-left: w1460 -> [w1465]
                      tunnel: string[] ["ARDUINO - ULTRASONIC", "READ ULTRASONIC", ""] -> [w1463] mode=indexing
                      n509 = Enqueue Element(queue=w1465, element=w1463) -> (queue out=w1464:refnum<queue>)  [unwired: 2 in, 2 out]
                    }
                  }
                }
                n510 = Or(x=w1448, y=w1447) -> (x .or. y?=w1450:bool)
                n511 = Select(t=State_Type_Definitions."True Stop" ("Enum"), s=w1447, f=State_Type_Definitions."Task 8B: MOVE TO BOX" ("Enum")) -> (s? t:f=w1444:T16)
                n512 = Select(t=w1444, s=w1450, f=State_Type_Definitions."Task 8A: RAISE ARM" ("Enum")) -> (s? t:f=w1449:T16)
              }
              frame "Exit" {
                n513 = for {
                  shift-right: [w1472] -> w1469
                  shift-left: w1466 -> [w1473]
                  tunnel: string[] ["STOP", "RESET ENCODERS", "RESET YAW", "ARDUINO MODE 0"] -> [w1471] mode=indexing
                  n514 = Enqueue Element(queue=w1473, element=w1471) -> (queue out=w1472:refnum<queue>)  [unwired: 2 in, 2 out]
                }
              }
            }
          }
          frame "Task 8B: MOVE TO BOX" {
            w1481 = u8 15 ("y")
            # ">>> yStepper command>>>"
            n515 = Less?(x=w1478, y=w1481) -> (x < y?=w1479:bool)
            n516 = Dequeue Element(queue=w1485, timeout in ms (-1)=w1484, error in (no error)=w1486) -> (element=w1483:T8)  [unwired: 3 out]